vi "transceiverRFID v1.vi"() -> ()   [LabVIEW 2015]
uses:
  <instrlib>/niUSRP/niUSRP Fetch Rx Data (CDB Cluster).vi
  <vilib>/measure/mamon.llb/Trigger Detection for 1 Channel.vi
  <vilib>/Waveform/WDTOps.llb/WDT Get Waveform Subset DBL.vi
  <instrlib>/niUSRP/niUSRP Write Tx Data (CDB).vi
  <vilib>/measure/NI_MAPro.lvlib
panel:
  out "error out 3":errorcluster
  in  "Parameters Query":T1 {"Session" items=["S0", "S1", "S2", "S3"]; "Sel" items=["All", "All2", "~SL", "SL"]; "M" items=["M=1", "M=2", "M=4", "M=8"]}
  in  "Symbol Rate [Hz]":dbl=500000.0 format="%#_13p"
  in  "Parameters Select":T2={"Target"=7, "Action"=0, "MemBank"=1, "truncate"=FALSE} {"MemBank" items=["00 RFU", "01 EPC", "10 TID", "11 User"]; "Action" items=["000", "001", "010", "011", "100", "101", "110", "111"]; "Target" items=["000 Inventoried (S0)", "001 Inventoried (S1)", "010 Inventoried (S2)", "011 Inventoried (S3)", "100 SL", "101 RFU", "110 RFU", "111 RFU"]}
  in  "Parameters Symbols":T3={"Tari"=8e-06, "PW"=0.5, "factor for \"1\" symbol"=0.5, "RTcal"=2.5, "TRcal"=3.0, "Delimiter"=1.4e-05} {"TRcal" min=1.1 max=3.0 step=0.1; "RTcal" min=2.5 max=3.0 step=0.1; "factor for \"1\" symbol" min=0.5 max=1.0 step=0.1; "PW" min=0.265 max=0.525 step=0.001; "Tari" format="%#_3p"}
  out "coerced IQ rate 2":dbl=100000.0 format="%#_6p"
  out "carrier frequency 3":dbl=100000.0 format="%#_6p"
  out "coerced gain 2":dbl format="%#_6f"
  in  "stop":bool
  out "Loop":i32
  out "RFID Pushed":bool
  in  "query":bool
  out "RN16 array":i32[](array[numeric])
  out "bits":i16[](graph)
  out "Wave Mag":dbl[](graph)
  out "ACK":bool
  in  "IQ rate 2":dbl=2000000.0 format="%#_6p"
  in  "carrier frequency 2":dbl=920000000.0 format="%#_6p"
  in  "gain 2":dbl format="%#_6f"
  in  "tx device names":refnum<k15>="192.168.20.13"
  in  "active antenna":string="RX2"
  in  "Channels":string(combo)="0"
  in  "timeout":dbl=10.0
  in  "number of samples":i64=2000000
  in  "Stop":bool
  out "Magnitude":cluster{"t0":dbl, "dt":dbl, "Y":dbl[]}(graph)={"t0"=22.57446071, "dt"=5e-07, "Y"=array[2000000 elements]}
  out "Triggered Signal":dynamicdata(graph)=[{"t0"=timestamp(16788727 s since 1904-01-01), "dt"=1.0, "Y"=array[700 elements], "attributes"=variant("NI_ChannelName"=variant(string "Trigger"))}]
  out "Portion Signal":dynamicdata(graph)
  out "start samples":dbl format="%.3g"
  out "duration samples":dbl format="%.3g"
  in  "start":i64=550 format="%.3g"
  in  "duration":dbl=180.0 format="%#_13g"
  out "RN16 waveform":i16[](graph)
  out "error out 2":errorcluster
  out "loop":i32
  out "trigger location":dbl format="%#_2g"
  out "Trigger":bool
  out "coerced gain":dbl format="%#_6f"
  out "coerced carrier frequency":dbl=100000.0 format="%#_6p"
  out "coerced IQ rate":dbl=100000.0 format="%#_6p"
  in  "gain":dbl format="%#_6f"
  in  "carrier frequency":dbl=920000000.0 format="%#_6p"
  in  "IQ rate":dbl=2000000.0 format="%#_6p"
  out "error out":errorcluster
  in  "device names":refnum<k15>="192.168.10.14"
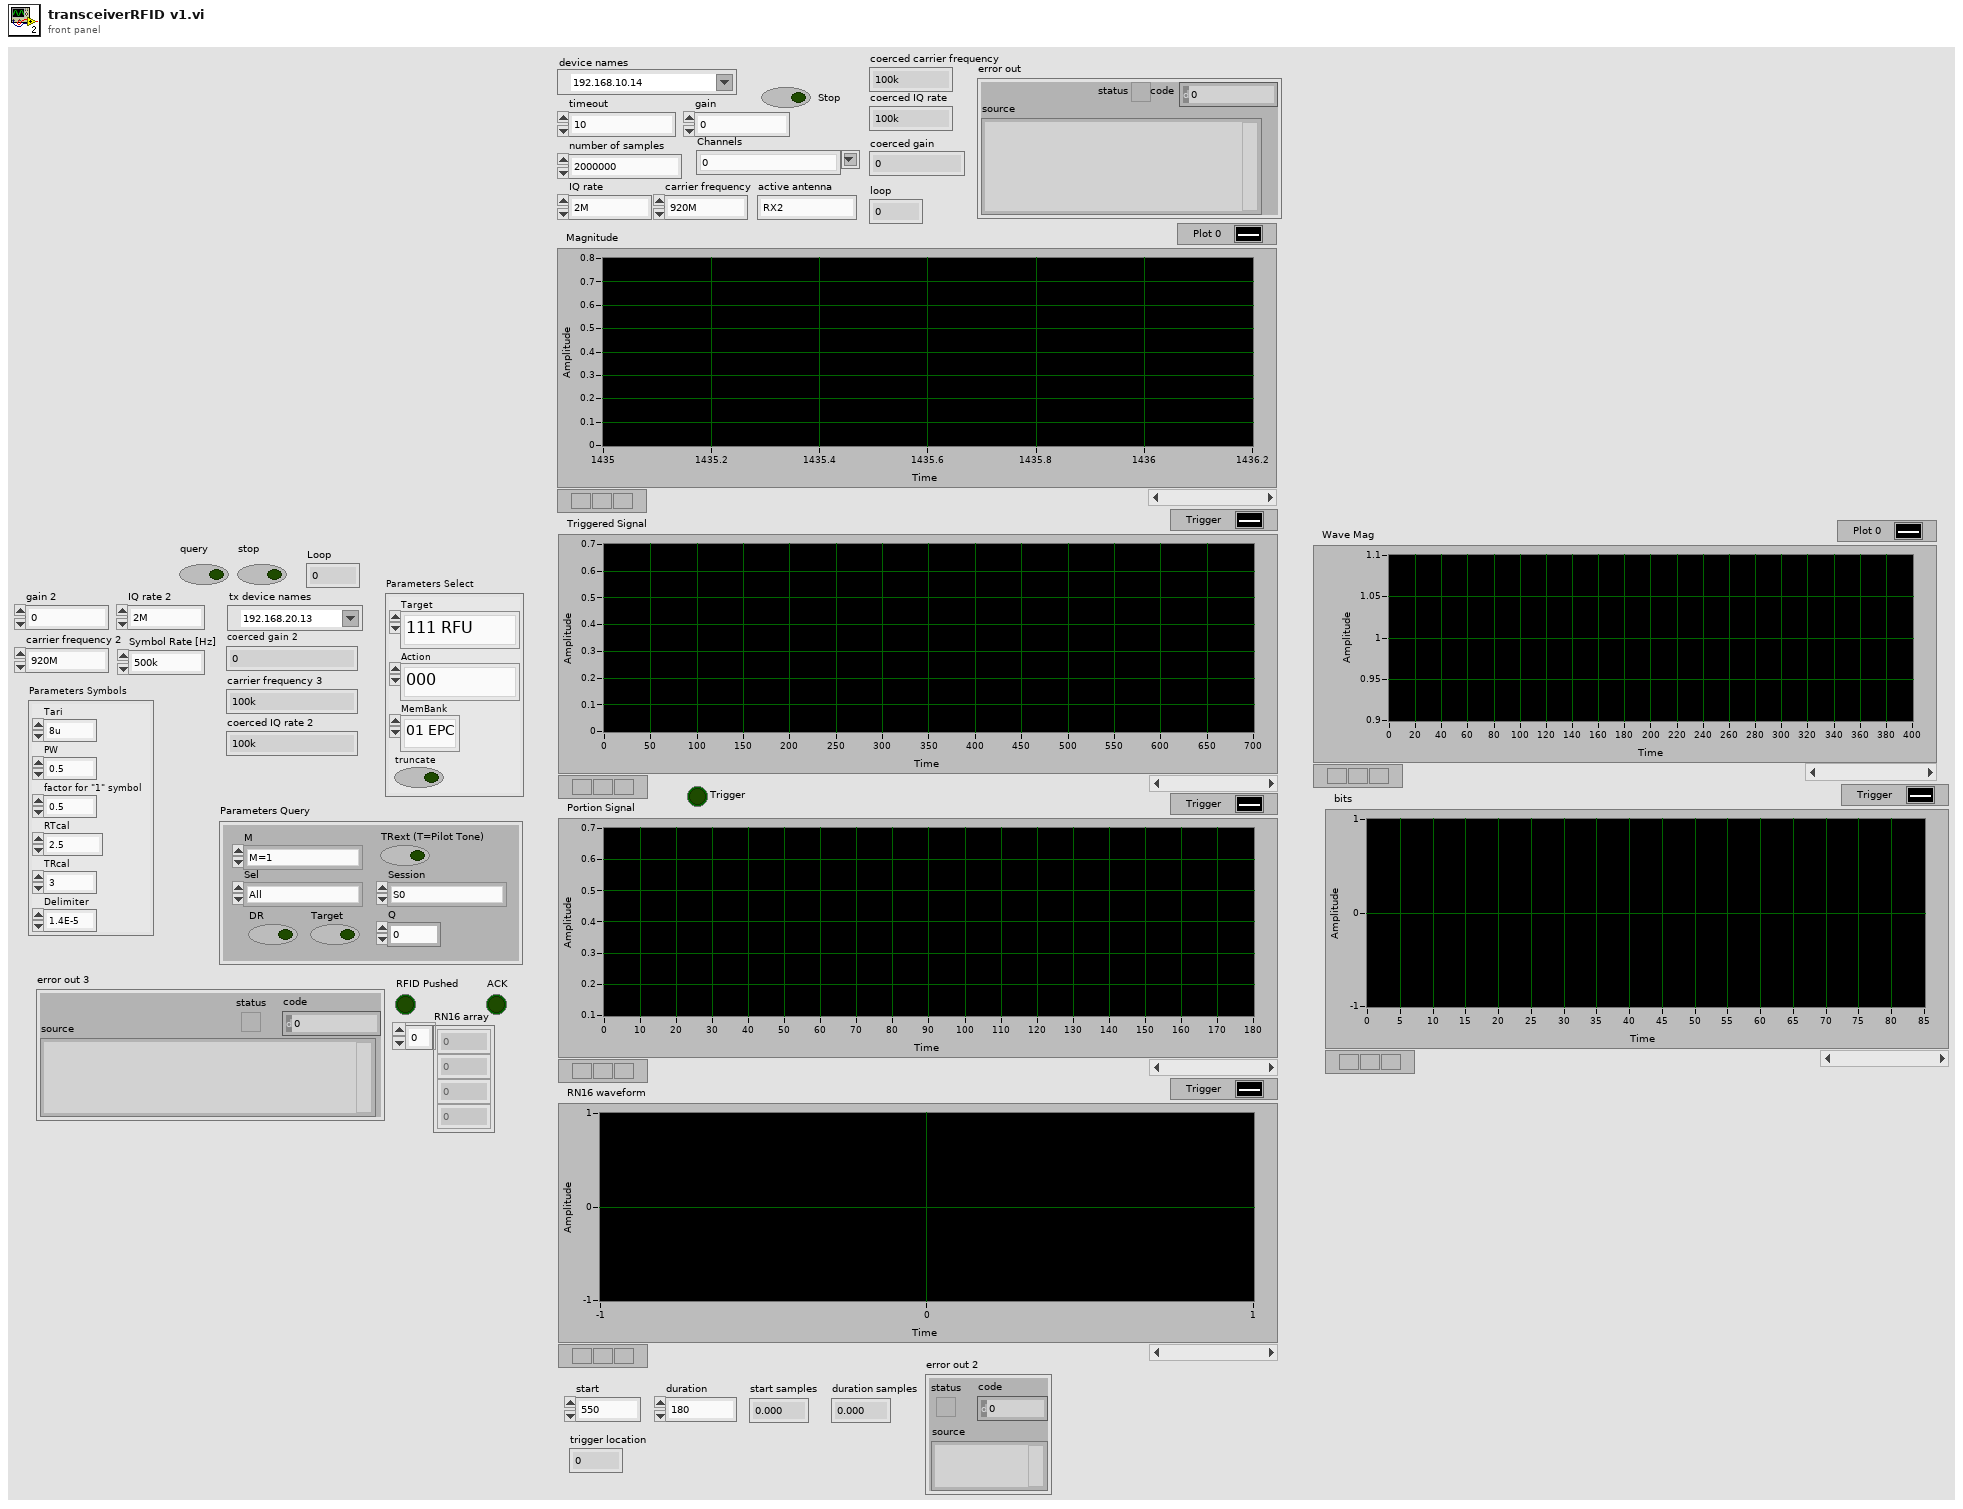
[diagram p1: front panel]
types:
  T1 = cluster{"DR":bool, "M":u16, "TRext (T=Pilot Tone)":bool, "Sel":u16, "Session":u16, "Q":u8, "Target":bool}
  T2 = cluster{"Target":u16, "Action":u16, "MemBank":u16, "truncate":bool}
  T3 = cluster{"Tari":dbl, "PW":dbl, "factor for \"1\" symbol":dbl, "RTcal":dbl, "TRcal":dbl, "Delimiter":dbl}
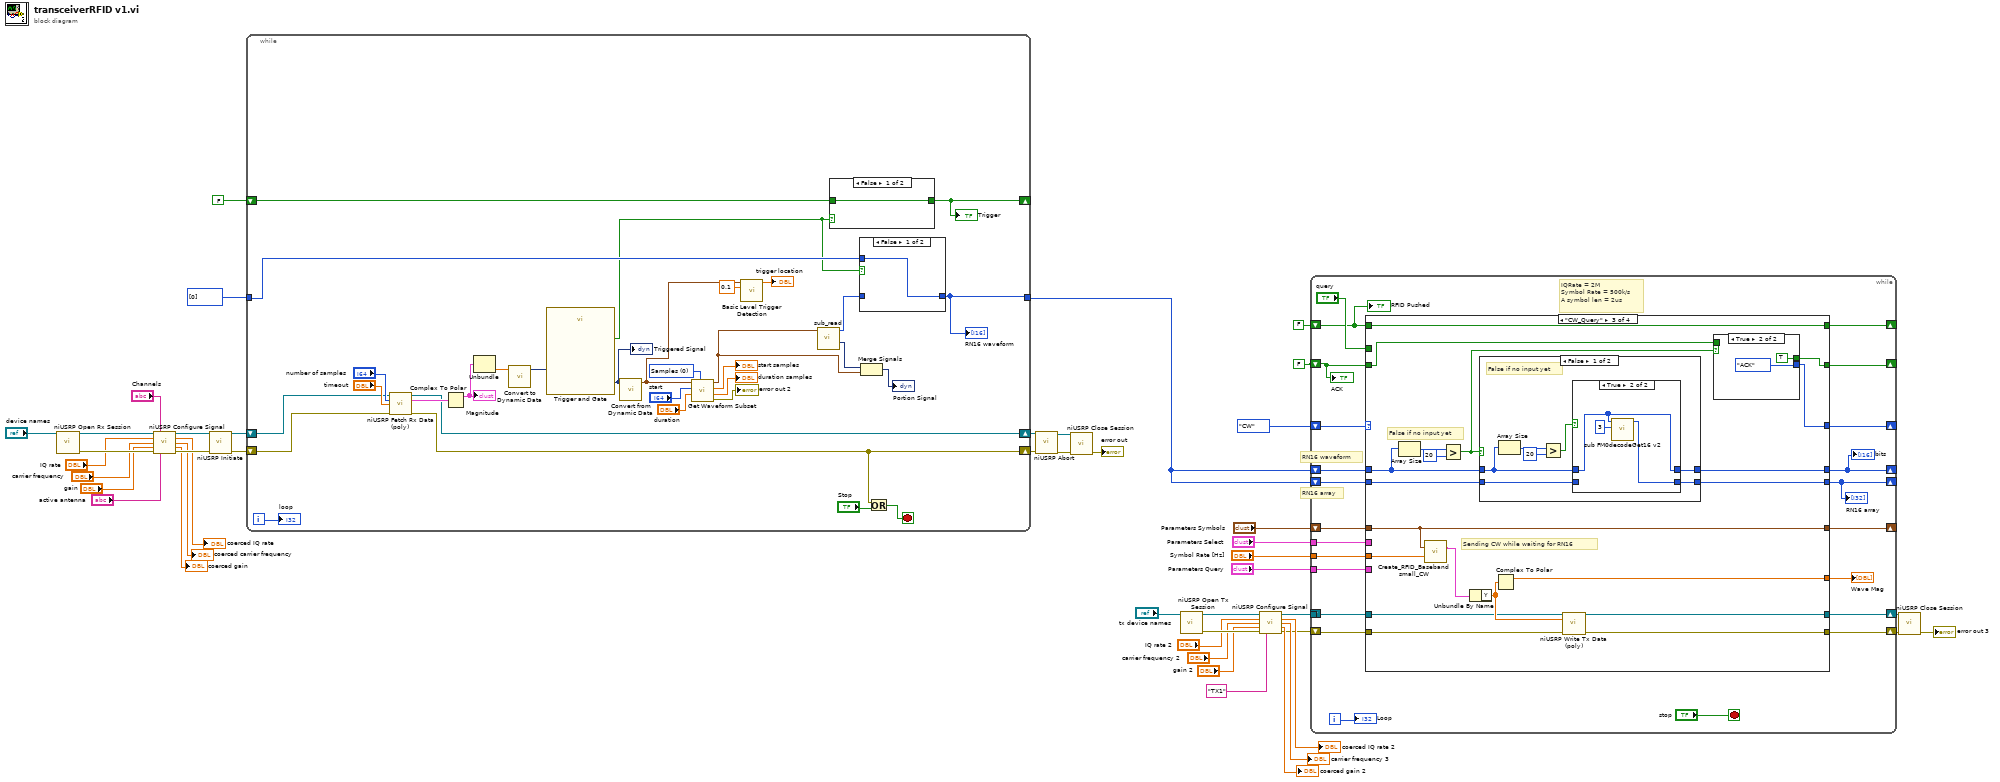
[diagram p0: block diagram]
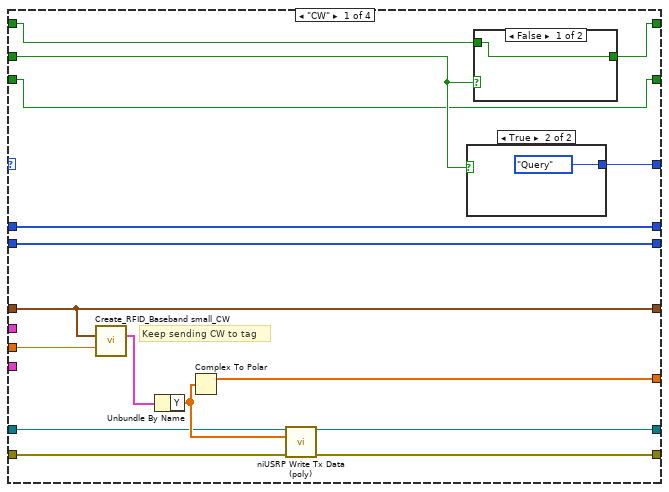
[diagram p2: hidden frame]
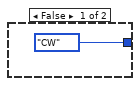
[diagram p4: hidden frame]
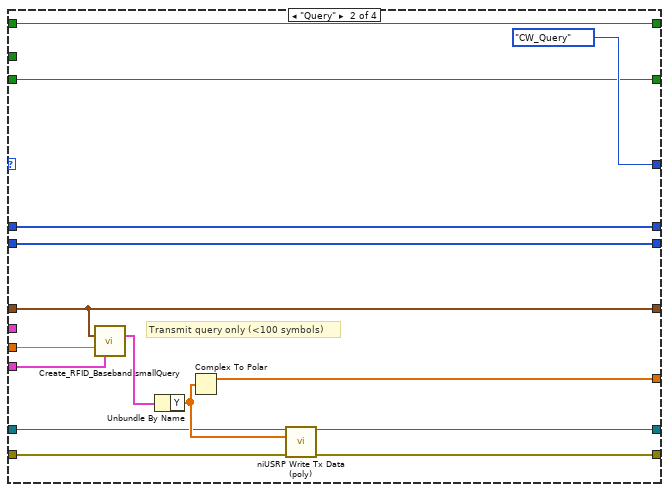
[diagram p5: hidden frame]
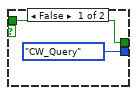
[diagram p6: hidden frame]
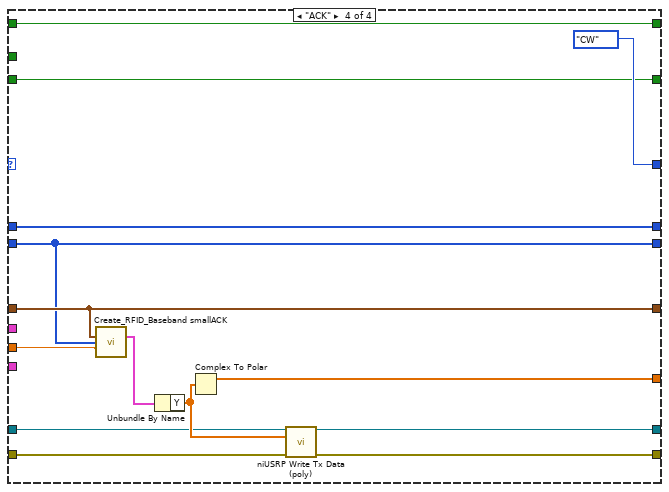
[diagram p9: hidden frame]
diagram:
  # "RN16 array"
  # "RN16 waveform"
  n1 = call <instrlib>:"niUSRP Open Rx Session.vi"("device names"="device names") -> ("session handle out"=w44:refnum<k15>, "error out"=w43:errorcluster)  [unwired: 13 in]
  n2 = call <instrlib>:"niUSRP Configure Signal.vi"("session handle"=w44, "channel list"="Channels", "IQ rate"="IQ rate", "carrier frequency"="carrier frequency", "gain"="gain", "error in (no error)"=w43, "active antenna"="active antenna") -> ("session handle out"=w42:refnum<k15>, "coerced IQ rate"=→"coerced IQ rate":dbl, "coerced carrier frequency"=→"coerced carrier frequency":dbl, "coerced gain"=→"coerced gain":dbl, "error out"=w41:errorcluster)  [unwired: 4 in]
  n3 = call <instrlib>:"niUSRP Initiate.vi"("session handle"=w42, "error in (no error)"=w41) -> ("session handle out"=w40:refnum<k15>, "error out"=w39:errorcluster)  [unwired: 12 in]
  n4 = while {
    shift-right: [w74] -> w38
    shift-left: w40 -> [w73]
    shift-right: [w57] -> w37
    shift-left: w39 -> [w72]
    shift-right: [w50] -> _
    shift-left: FALSE -> [w49]
    tunnel: i16[] [0] -> [w54]
    tunnel: [w48] -> w1
    i -> [w56]
    stop <- w69 stop-if-true
    w66 = u16 0 items=["Samples", "Relative Time"] ("start/duration format")
    n5 = call-poly <instrlib>:"niUSRP Fetch Rx Data (poly).vi"("session handle"=w73, "number of samples"="number of samples", "timeout"="timeout", "error in (no error)"=w72) -> ("session handle out"=w74:refnum<k15>, "data"=w75:cluster{"t0":dbl, "dt":dbl, "Y":cdb[]}, "error out"=w57:errorcluster)  [unwired: 8 in, 1 out]
    n6 = Complex To Polar(r * e^(i*theta)=w75) -> (r=w71:cluster{"t0":dbl, "dt":dbl, "Y":dbl[]})  [unwired: 1 out]
    "Magnitude" <- w71
    n7 = Unbundle(w71) -> ("Y"=w60:dbl[])  [unwired: 2 out]
    n8 = call "Convert to Dynamic Data"("Array"=w60) -> ("Dynamic Data Type"=w70:dynamicdata)  [unwired: 3 in]
    n9 = call "Trigger and Gate"("Signals"=w70) -> ("Triggered Signals"=w63:dynamicdata, "Data Available"=w47:bool)  [unwired: 7 in, 2 out]
    "Triggered Signal" <- w63
    n10 = call "Convert from Dynamic Data"("Dynamic Data Type"=w63) -> ("Waveform"=w51:waveform(dbl))  [unwired: 3 in]
    n11 = call-poly <vilib>:"Get Waveform Subset.vi"("start/duration format"=w66, "duration"="duration", "start samples/time"="start", "waveform in"=w51) -> ("error out"=→"error out 2":errorcluster, "actual duration"=→"duration samples":dbl, "actual start samples/time"=→"start samples":dbl, "waveform out"=w53:waveform(dbl))  [unwired: 2 in]
    n12 = call-poly <vilib>:"Basic Level Trigger Detection.vi"("signal in"=w51, "level"=0.1) -> ("trigger location"=→"trigger location":dbl)  [unwired: 11 in, 2 out]
    n13 = call "sub_read.vi"("Raw Signal"=w53) -> ("Digitized Sign"=w62:dynamicdata, "Bits"=w55:i16[])  [unwired: 6 in, 2 out]
    n14 = case shown="False" w47 {
      selector: w47 -> [_ w79]
      tunnel: [w78 w79] -> w50
      tunnel: w49 -> [w78 _]
      frame False {
      }
      frame True {
      }
    }
    "Trigger" <- w50
    n15 = case shown="False" w47 {
      tunnel: w55 -> [_ w81]
      tunnel: [w80 w81] -> w48
      tunnel: w54 -> [w80 _]
      frame False {
      }
      frame True {
      }
    }
    "RN16 waveform" <- w48
    n16 = Merge Signals(w62, w53) -> (→"Portion Signal":dynamicdata)
    n17 = Or(x=w57, y="Stop") -> (x .or. y?=w69:bool)
    "loop" <- w56
  }
  n18 = call <instrlib>:"niUSRP Abort.vi"("session handle"=w38, "error in (no error)"=w37) -> ("session handle out"=w36:refnum<k15>, "error out"=w35:errorcluster)  [unwired: 12 in]
  n19 = call <instrlib>:"niUSRP Close Session.vi"("session handle"=w36, "error in (no error)"=w35) -> ("error out"=→"error out":errorcluster)  [unwired: 13 in]
  n20 = call <instrlib>:"niUSRP Open Tx Session.vi"("device names"="tx device names") -> ("session handle out"=w4:refnum<k15>, "error out"=w23:errorcluster)  [unwired: 13 in]
  n21 = call <instrlib>:"niUSRP Configure Signal.vi"("session handle"=w4, "IQ rate"="IQ rate 2", "carrier frequency"="carrier frequency 2", "gain"="gain 2", "error in (no error)"=w23, "active antenna"="TX1") -> ("session handle out"=w10:refnum<k15>, "coerced IQ rate"=→"coerced IQ rate 2":dbl, "coerced carrier frequency"=→"carrier frequency 3":dbl, "coerced gain"=→"coerced gain 2":dbl, "error out"=w9:errorcluster)  [unwired: 5 in]
  n22 = while {
    tunnel: "Parameters Select" -> [w97]
    tunnel: "Parameters Query" -> [w95]
    tunnel: w10 -> [w102]
    shift-right: [w100] -> w8
    shift-left: w9 -> [w101]
    shift-right: [w99] -> w6
    shift-left: _ -> [_]
    shift-right: [w92] -> _
    shift-left: enum16{"CW", "Query", "CW_Query", "ACK"}."CW" -> [w103]
    shift-right: [w94] -> _
    shift-left: "Parameters Symbols" -> [w98]
    tunnel: "Symbol Rate [Hz]" -> [w96]
    shift-right: [w90] -> _
    shift-left: w1 -> [w91]
    shift-right: [w89] -> _
    shift-left: w1 -> [w88]
    shift-right: [w85] -> _
    shift-left: FALSE ("query") -> [w84]
    shift-right: [w82] -> _
    shift-left: FALSE ("query") -> [w83]
    i -> [w104]
    stop <- "stop" stop-if-true
    # "IQRate = 2M\nSymbol Rate = 500k/s\nA symbol len = 2us"
    n23 = case shown="\"CW_Query\"" w103 {
      tunnel: w102 -> [w119 w138 w158 w190]
      tunnel: w101 -> [w118 w137 w157 w189]
      tunnel: [w117 w136 w156 w188] -> w100
      tunnel: [w116 w135 w155 w187] -> w99
      tunnel: w98 -> [w114 w130 w146 w185]
      tunnel: w97 -> [_ _ _ _]
      tunnel: w96 -> [w113 w131 w145 w184]
      tunnel: w95 -> [_ w132 _ _]
      tunnel: [w114 w130 w146 w185] -> w94
      tunnel: [w115 w134 w154 w186] -> w87
      tunnel: [w111 enum16{"CW", "Query", "CW_Query", "ACK"}."CW_Query" w143 enum16{"CW", "Query", "CW_Query", "ACK"}."CW"] -> w92
      tunnel: "query" -> [w108 _ _ _]
      tunnel: w91 -> [w110 w129 w151 w181]
      tunnel: [w110 w129 w149 w181] -> w90
      tunnel: [w109 w128 w150 w182] -> w89
      tunnel: w88 -> [w109 w128 w148 w182]
      tunnel: [w107 w126 w142 w179] -> w85
      tunnel: w84 -> [w106 w126 w142 w179]
      tunnel: w83 -> [w105 w125 w141 w178]
      tunnel: [w105 w125 w140 w178] -> w82
      frame "CW" {
        # "Keep sending CW to tag"
        n24 = call "Create_RFID_Baseband small_CW.vi"("Parameters Symbols"=w114, "Symbol Rate [Hz]"=w113) -> ("complex waveform"=w112:cluster{"t0":dbl, "dt":dbl, "Y":cdb[]})  [unwired: 12 in, 1 out]
        n25 = Unbundle By Name(w112) -> ("Y"=w120:cdb[])
        n26 = Complex To Polar(r * e^(i*theta)=w120) -> (r=w115:dbl[])  [unwired: 1 out]
        n27 = call-poly <instrlib>:"niUSRP Write Tx Data (poly).vi"("session handle"=w119, "data"=w120, "error in (no error)"=w118) -> ("session handle out"=w116:refnum<k15>, "error out"=w117:errorcluster)  [unwired: 11 in]
        n28 = case shown="True" w108 {
          tunnel: [enum16{"CW", "Query", "CW_Query", "ACK"}."CW" enum16{"CW", "Query", "CW_Query", "ACK"}."Query"] -> w111
          frame False {
          }
          frame True {
          }
        }
        n29 = case shown="False" w108 {
          selector: w108 -> [_ w122]
          tunnel: [w121 w122] -> w107
          tunnel: w106 -> [w121 _]
          frame False {
          }
          frame True {
          }
        }
      }
      frame "Query" {
        # "Transmit query only (<100 symbols)"
        n30 = call "Create_RFID_Baseband smallQuery.vi"("Parameters Symbols"=w130, "Symbol Rate [Hz]"=w131, "Parameters Query"=w132) -> ("complex waveform"=w133:cluster{"t0":dbl, "dt":dbl, "Y":cdb[]})  [unwired: 11 in, 1 out]
        n31 = Unbundle By Name(w133) -> ("Y"=w139:cdb[])
        n32 = Complex To Polar(r * e^(i*theta)=w139) -> (r=w134:dbl[])  [unwired: 1 out]
        n33 = call-poly <instrlib>:"niUSRP Write Tx Data (poly).vi"("session handle"=w138, "data"=w139, "error in (no error)"=w137) -> ("session handle out"=w135:refnum<k15>, "error out"=w136:errorcluster)  [unwired: 11 in]
      }
      frame "CW_Query" {
        # "False if no input yet"
        # "Sending CW while waiting for RN16"
        n34 = Array Size(array=w151) -> (size(s)=w152:i32)
        n35 = call "Create_RFID_Baseband small_CW.vi"("Parameters Symbols"=w146, "Symbol Rate [Hz]"=w145) -> ("complex waveform"=w147:cluster{"t0":dbl, "dt":dbl, "Y":cdb[]})  [unwired: 12 in, 1 out]
        n36 = Greater?(x=w152, y=20) -> (0:w144:bool)
        n37 = Unbundle By Name(w147) -> ("Y"=w159:cdb[])
        n38 = case shown="False" w144 {
          tunnel: [w167 w177] -> w149
          tunnel: w151 -> [w164 w177]
          tunnel: [w166 w176] -> w150
          tunnel: w148 -> [w165 w176]
          frame False {
            # "False if no input yet"
            n39 = Array Size(array=w164) -> (size(s)=w170:i32)
            n40 = Greater?(x=w170, y=20) -> (0:w168:bool)
            n41 = case shown="True" w168 {
              tunnel: w164 -> [w172 w173]
              tunnel: [w172 w173] -> w167
              tunnel: [w171 w175] -> w166
              tunnel: w165 -> [w171 _]
              frame False {
              }
              frame True {
                n42 = call "sub FM0decodeGet16 v2.vi"("threshold"=3, "RN16 waveform"=w173) -> ("RN16 array"=w175:i32[])  [unwired: 9 in]
              }
            }
          }
          frame True {
          }
        }
        n43 = Complex To Polar(r * e^(i*theta)=w159) -> (r=w154:dbl[])  [unwired: 1 out]
        n44 = call-poly <instrlib>:"niUSRP Write Tx Data (poly).vi"("session handle"=w158, "data"=w159, "error in (no error)"=w157) -> ("session handle out"=w155:refnum<k15>, "error out"=w156:errorcluster)  [unwired: 11 in]
        n45 = case shown="True" w144 {
          tunnel: [enum16{"CW", "Query", "CW_Query", "ACK"}."CW_Query" enum16{"CW", "Query", "CW_Query", "ACK"}."ACK"] -> w143
          tunnel: w141 -> [w160 _]
          tunnel: [w160 TRUE ("query")] -> w140
          frame False {
          }
          frame True {
          }
        }
      }
      frame "ACK" {
        n46 = call "Create_RFID_Baseband smallACK.vi"("Parameters Symbols"=w185, "RN16 array"=w182, "Symbol Rate [Hz]"=w184) -> ("complex waveform"=w183:cluster{"t0":dbl, "dt":dbl, "Y":cdb[]})  [unwired: 11 in, 1 out]
        n47 = Unbundle By Name(w183) -> ("Y"=w191:cdb[])
        n48 = Complex To Polar(r * e^(i*theta)=w191) -> (r=w186:dbl[])  [unwired: 1 out]
        n49 = call-poly <instrlib>:"niUSRP Write Tx Data (poly).vi"("session handle"=w190, "data"=w191, "error in (no error)"=w189) -> ("session handle out"=w187:refnum<k15>, "error out"=w188:errorcluster)  [unwired: 11 in]
      }
    }
    "RN16 array" <- w89
    "bits" <- w90
    "Wave Mag" <- w87
    "Loop" <- w104
    "RFID Pushed" <- w84
    "ACK" <- w83
  }
  n50 = call <instrlib>:"niUSRP Close Session.vi"("session handle"=w6, "error in (no error)"=w8) -> ("error out"=→"error out 3":errorcluster)  [unwired: 13 in]
